vi "View_series_FITS.vi"() -> ()   [LabVIEW 2017] (continued)
, 109.0, 70.0, 62.0, 60.0, 158.0, 79.0, 92.0, 161.0, 66.0, 67.0, 78.0, 96.0, 109.0, 51.0, 173.0, 108.0, 147.0, 183.0, 74.0, 94.0, 120.0, 80.0, 134.0, 89.0, 56.0, -16.0, 94.0, 90.0, 26.0, 124.0, 88.0, 88.0, 82.0, 56.0, 67.0, 93.0, 104.0, 82.0, 121.0, 84.0, 115.0, 46.0, 101.0, 77.0, 20.0, 108.0, 66.0, 88.0, 74.0, 66.0, 126.0, 130.0, 33.0, 104.0, 88.0, 129.0, 93.0, 91.0, 78.0, 31.0, 129.0, 73.0, 40.0, 105.0, 78.0, 80.0, 99.0, 114.0, 52.0, 108.0, 54.0, 63.0, 88.0, 99.0, 96.0, 116.0, 92.0, 84.0, 146.0, 71.0, 65.0, 106.0, 107.0, 133.0, 136.0, 109.0, 113.0, 73.0, 41.0, 90.0, 175.0, 81.0, 107.0, 134.0, 135.0, 104.0, 85.0, 121.0, 80.0, 109.0, 166.0, 147.0, 133.0, 117.0, 132.0, 154.0, 125.0, 124.0, 150.0, 200.0, 161.0, 126.0, 171.0, 266.0, 175.0, 177.0, 301.0, 265.0, 149.0, 143.0, 185.0, 299.0, 158.0, 120.0, 119.0, 255.0, 290.0, 245.0, 254.0, 309.0, 205.0, 224.0, 379.0, 343.0, 303.0, 316.0, 480.0, 435.0, 437.0, 410.0, 625.0, 508.0, 572.0, 872.0, 768.0, 1180.0, 1554.0, 1463.0, 1204.0, 1306.0, 1805.0, 1380.0, 1684.0, 1665.0, 2388.0, 1898.0, 1150.0, 1765.0, 1211.0, 1278.0, 1008.0, 755.0, 628.0, 505.0, 380.0, 509.0, 498.0, 455.0, 590.0, 512.0, 447.0, 285.0, 518.0, 373.0, 347.0, 317.0, 322.0, 335.0, 182.0, 205.0, 264.0, 179.0, 156.0, 290.0, 216.0, 180.0, 107.0, 66.0, 97.0, 100.0, 130.0, 148.0, 131.0, 97.0, 112.0, 125.0, 104.0, 157.0, 124.0, 154.0, 66.0, 113.0, 70.0, 83.0, 127.0, 97.0, 133.0, 80.0, 106.0, 69.0, 123.0, 128.0, 87.0, 116.0, 106.0, 124.0, 96.0, 61.0, 112.0, 69.0, 77.0, 43.0, 88.0, 138.0, 109.0, 102.0, 48.0, 56.0, 88.0, 44.0, 80.0, 106.0, 84.0, 59.0, 88.0, 72.0, 115.0, 82.0, 22.0, 57.0, 78.0, 100.0, 84.0, 79.0, 125.0, 91.0, 85.0, 106.0, -2.0, 0.0, -10.0, 1.0, 2.0, 0.0, 12.0, -14.0, 0.0, 186.0, 188.0, 100.0, 148.0, 52.0, 86.0, 80.0, 90.0, 64.0, 98.0, 80.0, 106.0, 102.0, 100.0, 136.0, 90.0, 40.0, 134.0, 74.0, 64.0, 120.0, 74.0, 134.0, 96.0, 62.0, 80.0, 102.0, 106.0, 58.0, 122.0, 100.0, 70.0, 126.0, 74.0, 80.0, 112.0, 44.0, 94.0, 118.0, 80.0, 114.0, 144.0, 86.0, 72.0, 102.0, 128.0, 88.0, 120.0, 94.0, 136.0, 146.0, 122.0, 134.0, 106.0, 160.0, 174.0, 204.0, 276.0, 280.0, 200.0, 334.0, 240.0, 220.0, 342.0, 302.0, 330.0, 250.0, 354.0, 268.0, 258.0, 236.0, 158.0, 194.0, 144.0, 218.0, 134.0, 130.0, 116.0, 80.0, 110.0, 126.0, 130.0, 120.0, 98.0, 130.0, 100.0, 148.0, 106.0, 98.0, 110.0, 128.0, 98.0, 72.0, 104.0, 108.0, 132.0, 104.0, 108.0, 66.0, 204.0, 104.0, 104.0, 114.0, 86.0, 104.0, 38.0, 128.0, 104.0, 100.0, 122.0, 72.0, 72.0, 122.0, 156.0, 140.0, 132.0, 148.0, 86.0, 72.0, 106.0, 122.0, 140.0, 68.0, 82.0, 110.0, 80.0, 130.0, 88.0, 98.0, 112.0, 136.0, 138.0, 224.0, 86.0, 82.0, 104.0, 36.0, 86.0, 82.0, 100.0, 108.0, 108.0, 140.0, 100.0, 162.0, 118.0, 92.0, 100.0, 134.0, 68.0, 114.0, 102.0, 154.0, 84.0, 96.0, 178.0, 116.0, 224.0, 132.0, 78.0, 166.0, 130.0, 142.0, 114.0, 144.0, 84.0, 76.0, 148.0, 278.0, 122.0, 208.0, 172.0, 174.0, 132.0, 82.0, 94.0, 124.0, 202.0, 134.0, 170.0, 176.0, 156.0, 160.0, 130.0, 260.0, 244.0, 164.0, 208.0, 330.0, 324.0, 286.0, 462.0, 460.0, 358.0, 298.0, 422.0, 496.0, 368.0, 356.0, 492.0, 636.0, 582.0, 912.0, 590.0, 728.0, 960.0, 1122.0, 1322.0, 1146.0, 1358.0, 1412.0, 1668.0, 1750.0, 1348.0, 1494.0, 1784.0, 1630.0, 2430.0, 2424.0, 2260.0, 2330.0, 2126.0, 1934.0, 2190.0, 1808.0, 2816.0, 1314.0, 1562.0, 944.0, 1196.0, 1498.0, 1230.0, 1150.0, 930.0, 856.0, 894.0, 738.0, 720.0, 714.0, 570.0, 602.0, 560.0, 482.0, 432.0, 392.0, 480.0, 290.0, 352.0, 378.0, 292.0, 252.0, 352.0, 286.0, 236.0, 280.0, 258.0, 186.0, 266.0, 310.0, 282.0, 212.0, 342.0, 232.0, 222.0, 208.0, 230.0, 174.0, 280.0, 196.0, 138.0, 232.0, 256.0, 132.0, 154.0, 166.0, 262.0, 220.0, 184.0, 130.0, 204.0, 150.0, 124.0, 158.0, 210.0, 190.0, 94.0, 154.0, 146.0, 126.0, 148.0, 110.0, 152.0, 198.0, 152.0, 168.0, 118.0, 80.0, 76.0, 124.0, 150.0, 130.0, 102.0, 122.0, 128.0, 162.0, 136.0, 96.0, 232.0, 154.0, 102.0, 150.0, 102.0, 96.0, 114.0, 118.0, 106.0, 166.0, 118.0, 144.0, 154.0, 200.0, 140.0, 54.0, 112.0, 106.0, 142.0, 108.0, 170.0, 138.0, 122.0, 120.0, 96.0, 92.0, 156.0, 120.0, 196.0, 130.0, 144.0, 138.0, 164.0, 64.0, 200.0, 166.0, 212.0, 162.0, 206.0, 148.0, 134.0, 128.0, 152.0, 180.0, 164.0, 194.0, 180.0, 168.0, 102.0, 146.0, 180.0, 152.0, 228.0, 132.0, 158.0, 126.0, 130.0, 170.0, 130.0, 128.0, 168.0, 92.0, 164.0, 164.0, 96.0, 130.0, 118.0, 104.0, 112.0, 162.0, 184.0, 140.0, 232.0, 68.0, 72.0, 146.0, 108.0, 96.0, 102.0, 114.0, 108.0, 152.0, 132.0, 124.0, 82.0, 126.0, 116.0, 96.0, 128.0, 48.0, 86.0, 96.0, 62.0, 156.0, 126.0, 118.0, 132.0, 150.0, 128.0, 64.0, 54.0, 44.0, 52.0, 76.0, 112.0, 156.0, 120.0, 138.0, 136.0, 128.0, 114.0, 86.0, 80.0, 94.0, 150.0, 110.0, 164.0, 64.0, 110.0, 74.0, 130.0, 114.0, 96.0, 114.0, 166.0, 144.0, 64.0, 98.0, 70.0, 92.0, 102.0, 130.0, 90.0, 82.0, 80.0, 68.0, 166.0, 84.0, 32.0, 100.0, 82.0, 110.0, 144.0, 72.0, 78.0, 208.0, 102.0, 144.0, 96.0, 106.0, 56.0, 96.0, 110.0, 82.0, 68.0, 112.0, 168.0, 124.0, 124.0, 42.0, 78.0, 114.0, 82.0, 134.0, 142.0, 122.0, 124.0, 84.0, 116.0, 96.0, 86.0, 106.0, 70.0, 92.0, 124.0, 142.0, 144.0, 80.0, 84.0, 70.0, 106.0, 152.0, 92.0, 50.0, 110.0, 90.0, 100.0, 98.0, 110.0, 82.0, 78.0, 94.0, 80.0, 88.0, 90.0, 90.0, 46.0, 86.0, 122.0, 60.0, 65.0, 120.0, 78.0, 80.0, 77.0, 88.0, 124.0, 98.0, 163.0, 94.0, 140.0, 84.0, 86.0, 152.0, 73.0, 111.0, 73.0, 77.0, 103.0, 96.0, 91.0, 163.0, 90.0, 96.0, 172.0, 94.0, 130.0, 88.0, 119.0, 47.0, 82.0, 135.0, 116.0, 84.0, 148.0, 68.0, 121.0, 57.0, 162.0, 95.0, 105.0, 51.0, 67.0, 108.0, 102.0, 210.0, 68.0, 109.0, 136.0, 50.0, 188.0, 188.0, 146.0, 132.0, 106.0, 111.0, 56.0, 113.0, 101.0, 108.0, 79.0, 134.0, 89.0, 102.0, 111.0, 92.0, 140.0, 120.0, 56.0, 112.0, 147.0, -31.0, 104.0, 125.0, 15.0, 104.0, 84.0, 77.0, 104.0, 52.0, 121.0, 145.0, 78.0, 125.0, 158.0, 120.0, 78.0, 129.0, 115.0, 102.0, 104.0, 96.0, 151.0, 107.0, 80.0, 108.0, 114.0, 144.0, 69.0, 100.0, 114.0, 137.0, 76.0, 137.0, 66.0, 148.0, 56.0, 156.0, 142.0, 121.0, 130.0, 135.0, 164.0, 120.0, 93.0, 153.0, 116.0, 121.0, 136.0, 90.0, 93.0, 115.0, 44.0, 141.0, 95.0, 96.0, 132.0, 144.0, 209.0, 99.0, 70.0, 128.0, 143.0, 62.0, 141.0, 140.0, 70.0, 107.0, 50.0, 63.0, 151.0, 118.0, 151.0, 71.0, 101.0, 83.0, 109.0, 111.0, 158.0, 86.0, 133.0, 175.0, 154.0, 129.0, 93.0, 76.0, 142.0, 88.0, 38.0, -30.0, 61.0, 117.0, 125.0, 106.0, 86.0, 140.0, 112.0, 165.0, 131.0, 156.0, 132.0, 115.0, 156.0, 146.0, 169.0, 92.0, 111.0, 115.0, 120.0, 116.0, 94.0, 64.0, 80.0, 118.0, 141.0, 43.0, 83.0, 92.0, 132.0, 127.0, 141.0, 119.0, 101.0, 89.0, 92.0, 141.0, 105.0, 141.0, 93.0, 105.0, 95.0, 155.0, 127.0, 85.0, 221.0, 149.0, 131.0, 140.0, 87.0, 56.0, 98.0, 121.0, 23.0, 102.0, 93.0, 101.0, 57.0, 79.0, 116.0, 29.0, 124.0, 63.0, 116.0, 172.0, 101.0, 108.0, 129.0, 121.0, 126.0, 74.0, 78.0, 162.0, 60.0, 78.0, 96.0, 117.0, 103.0, 146.0, 179.0, 256.0, 172.0, 179.0, 39.0, 59.0, 106.0, 77.0, 112.0, 136.0, 133.0, 105.0, 168.0, 166.0, 133.0, 147.0, 172.0, 135.0, 95.0, 76.0, 148.0, 63.0, 145.0, 182.0, 90.0, 107.0, 118.0, 150.0, 84.0, 78.0, 119.0, 158.0, 85.0, 53.0, 160.0, 134.0, 120.0, 134.0, 126.0, 229.0, 125.0, 128.0, 101.0, 132.0, 175.0, 127.0, 202.0, 151.0, 130.0, 108.0, 189.0, 157.0, 112.0, 231.0, 149.0, 193.0, 107.0, 143.0, 151.0, 138.0, 147.0, 123.0, 118.0, 276.0, 96.0, 127.0, 130.0, 151.0, 125.0, 114.0, 119.0, 106.0, 151.0, 129.0, 184.0, 125.0, 89.0, 166.0, 142.0, 133.0, 113.0, 96.0, 143.0, 167.0, 143.0, 216.0, 158.0, 80.0, 216.0, 44.0, 79.0, 123.0, 96.0, 140.0, 153.0, 118.0, 127.0, 119.0, 76.0, 146.0, 97.0, 115.0, 120.0, 129.0, 144.0, 80.0, 105.0, 98.0, 124.0, 111.0, 97.0, 138.0, 124.0, 128.0, 86.0, 113.0, 127.0, 123.0, 128.0, 108.0, 147.0, 108.0, 93.0, 113.0, 59.0, 134.0, 155.0, 108.0, 164.0, 109.0, 127.0, 182.0, 110.0, 180.0, 118.0, 66.0, 88.0, 161.0, 97.0, 175.0, 197.0, 197.0, 157.0, 133.0, 100.0, 130.0, 112.0, 110.0, 200.0, 185.0, 183.0, 144.0, 164.0, 140.0, 114.0, 147.0, 181.0, 267.0, 197.0, 172.0, 157.0, 236.0, 161.0, 209.0, 220.0, 262.0, 210.0, 318.0, 283.0, 173.0, 312.0, 252.0, 237.0, 112.0, 367.0, 343.0, 226.0, 352.0, 311.0, 292.0, 488.0, 539.0, 467.0, 476.0, 430.0, 523.0, 361.0, 558.0, 542.0, 569.0, 788.0, 668.0, 948.0, 709.0, 1137.0, 906.0, 1089.0, 1344.0, 1373.0, 1444.0, 1630.0, 1584.0, 2442.0, 1776.0, 1876.0, 1835.0, 1217.0, 1901.0, 1929.0, 1557.0, 1665.0, 1196.0, 1374.0, 1362.0, 1216.0, 1006.0, 1012.0, 1299.0, 1141.0, 654.0, 905.0, 969.0, 719.0, 570.0, 635.0, 485.0, 693.0, 490.0, 414.0, 377.0, 321.0, 370.0, 372.0, 263.0, 284.0, 197.0, 143.0, 267.0, 263.0, 247.0, 202.0, 293.0, 241.0, 242.0, 147.0, 142.0, 184.0, 191.0, 164.0, 151.0, 160.0, 115.0, 127.0, 178.0, 180.0, 105.0, 221.0, 139.0, 71.0, 130.0, 146.0, 111.0, 93.0, 148.0, 56.0, 56.0, 104.0, 75.0, 113.0, 65.0, 5.0, -8.0, 9.0, -1.0]
  in  "pattern (all files)":string="*.fits"
  in  "path":path=path "C:/DATA/20110304/series_focus_IN_150um"
  out "Input File:":path=path "C:/DATA/20110304/series_focus_IN_150um/111030412.5622.fits"
  out "Image":dbl[][](graph)
  # "A1"
  # "RIGHT"
  # "TOP"
  # "A2"
  # "A3"
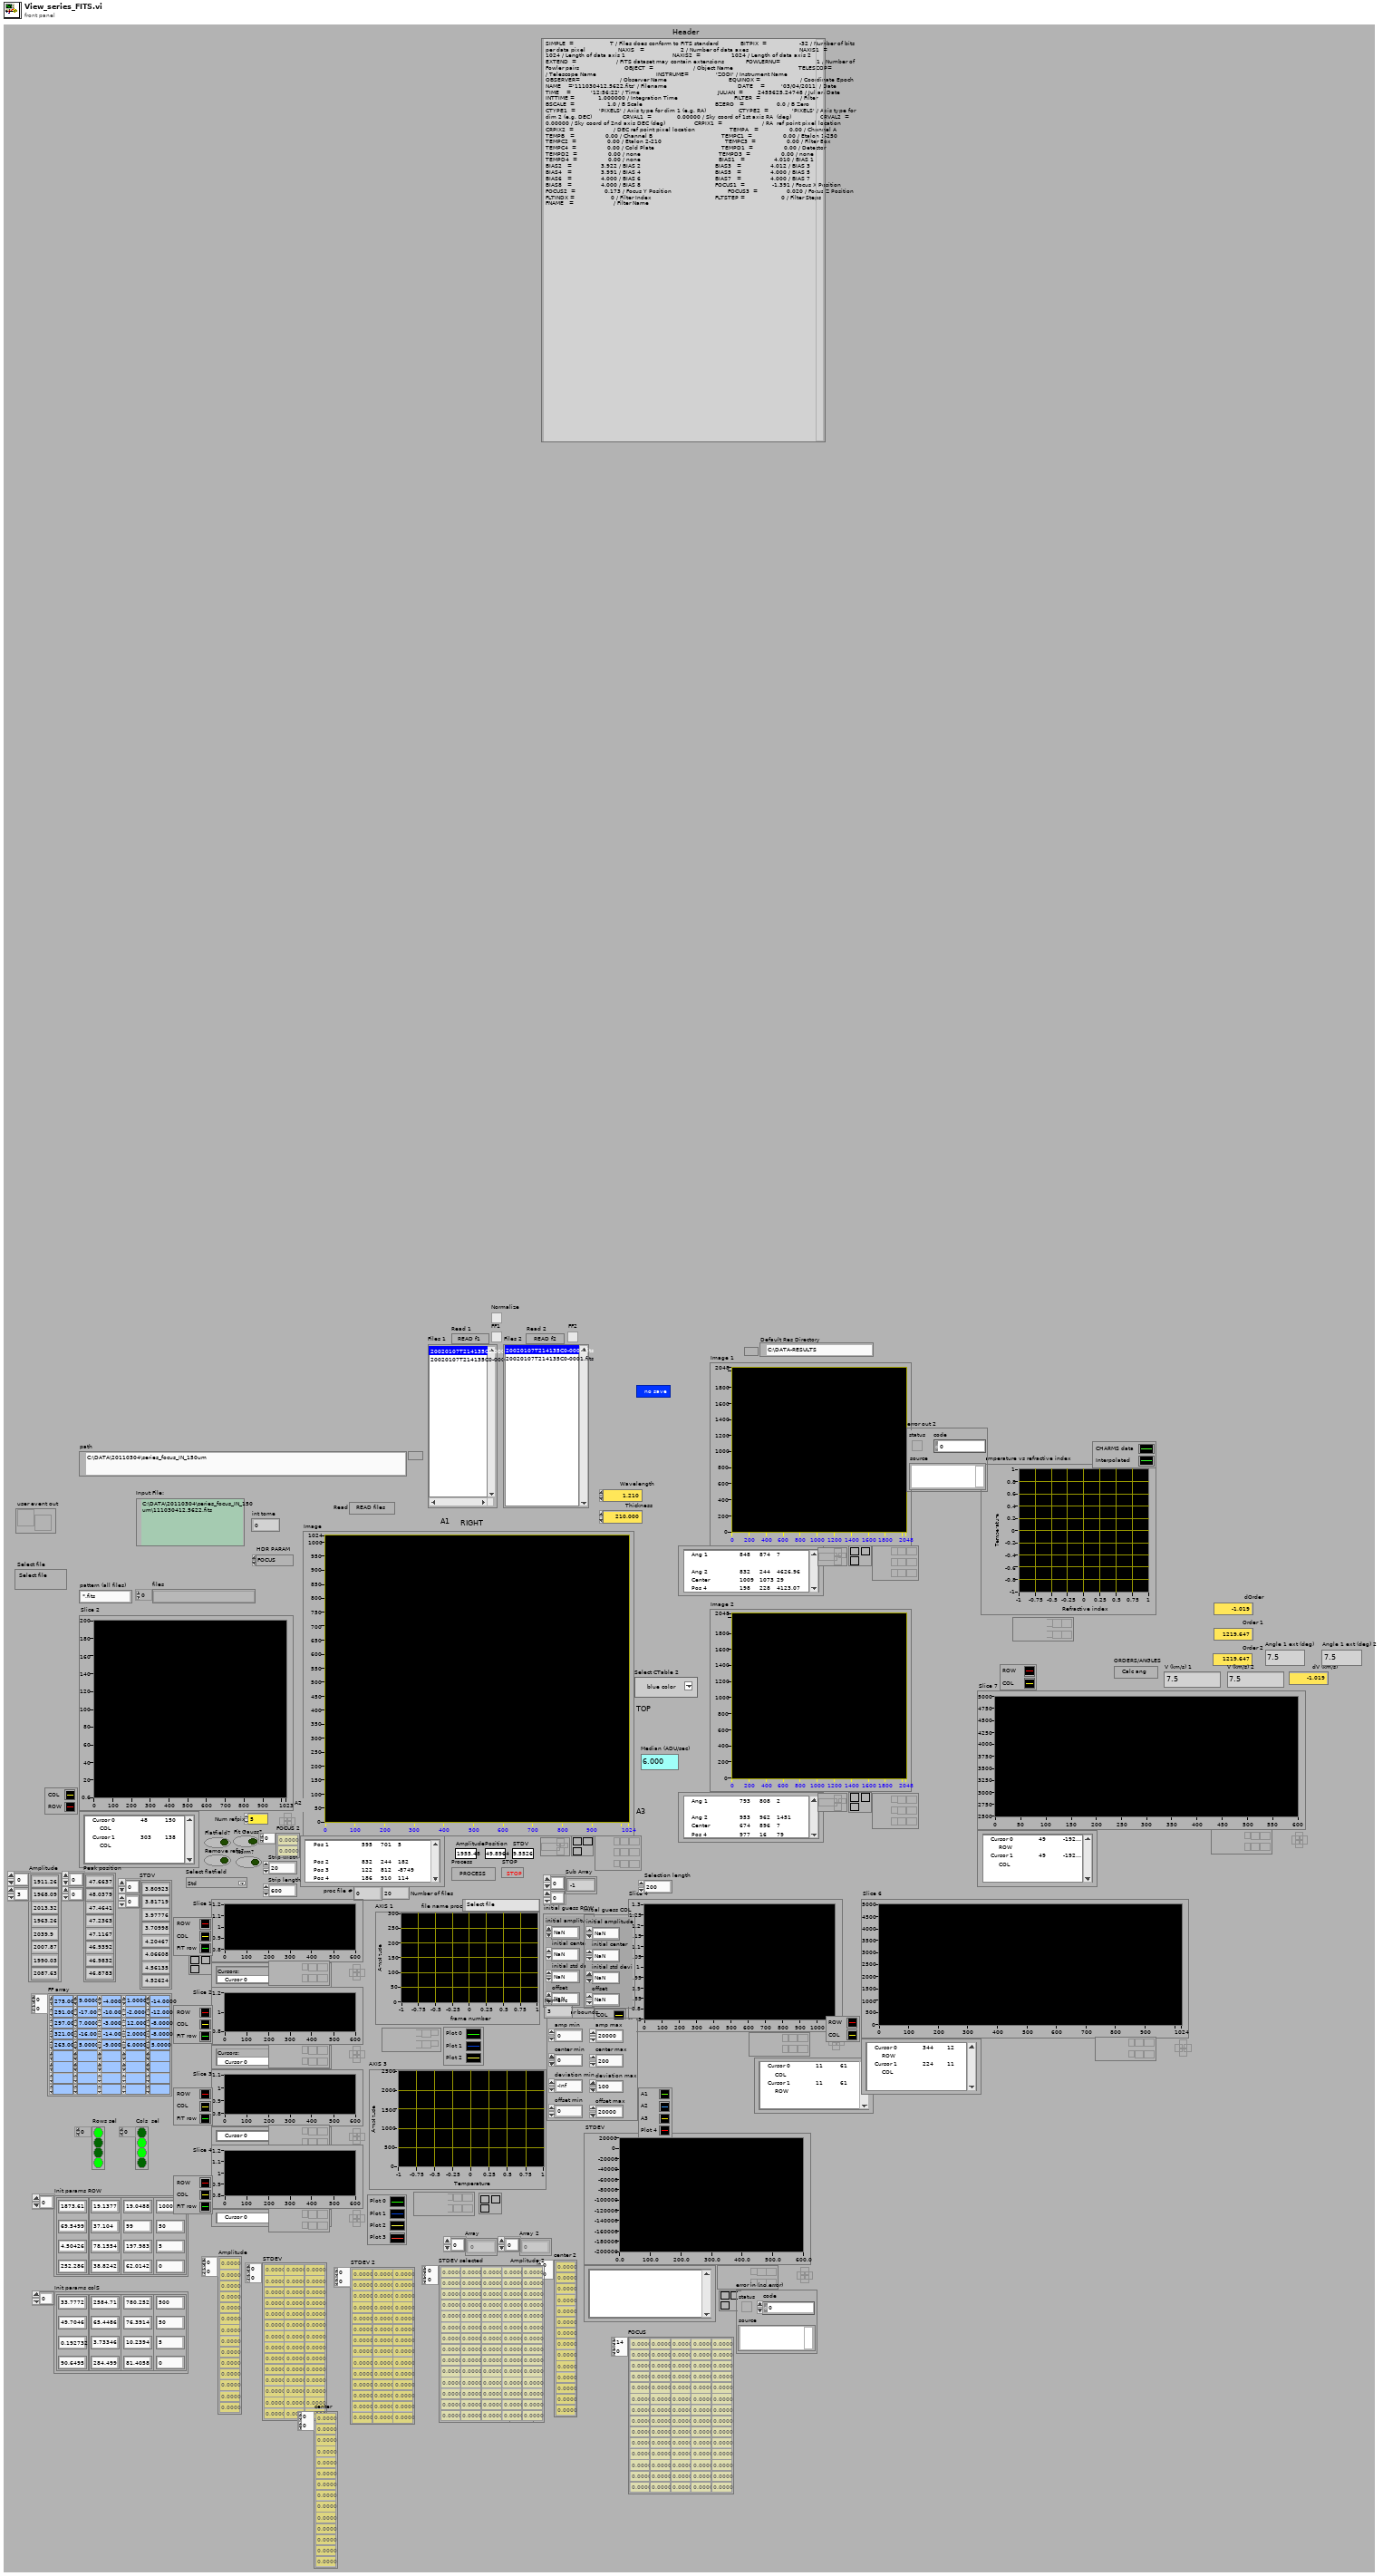
[diagram p1: front panel]
types:
  T1 = typedef "Color Table .ctl" = u16
  T2 = cluster{"initial amplitude":dbl, "initial center":dbl, "initial std devi":dbl, "offset":dbl}[]
  T3 = cluster{"initial amplitude":dbl, "initial center":dbl, "initial std devi":dbl, "offset":dbl}
  T4 = cluster{"amp min":dbl, "amp max":dbl, "center min":dbl, "center max":dbl, "deviation min":dbl, "deviation max":dbl, "offset min":dbl, "offset max":dbl}
  T5 = typedef "RIMAS Control Configuration.ctl" = cluster{"password":string, "Thermal Settings":T6, "Detector Config":T7, "Filter Wheel Config":T10}
  T6 = typedef "Thermal Control Configuration.ctl" = cluster{"Port":refnum<visa-resource-name>, "Recording Interval":dbl}
  T7 = typedef "RIMAS Detector Config.ctl" = cluster{"Detector":u16, "Offsets 0":u16[], "Detector Computer":T8, "FITS hdr template0":path, "FITS hdr template1":path, "FITS Data File Path":path, "FITS Detector Settings":T9, "Offsets 1":u16[]}
  T8 = typedef "RIMAS Detector Server Config.ctl" = cluster{"Machine":string, "Port":u16, "Password":string, "FITS File Path":string, "Header Path":string}
  T9 = typedef "RIMAS Observation Config.ctl" = cluster{"Exp Time Short":dbl, "# of Frames":dbl, "Exp Time Long":dbl, "# of Groups":dbl, "Object Name":string, "Object":string, "Obs Type":string, "Image Type":string, "Observer":string, "Observer Affiliation":string}
  T10 = typedef "RIMAS Filter Wheel Configuration.ctl" = cluster{"Port":refnum<visa-resource-name>, "Filters":T11, "Move parameters":T16, "Steps to move to filters CW":u16[], "delay before \nstop (ms)":u32}
  T11 = typedef "RIMAS Filter Wheel Positions Cluster.ctl" = cluster{"Filter 1":T12, "Filter 2":T13, "FP Filter":T14, "Slit":T15}
  T12 = typedef "RIMAS Filter Wheel enum Filter 1.ctl" = enum16{"H", "K", "Open", "Closed", "Low Res", "Hi Res"}
  T13 = typedef "RIMAS Filter Wheel enum Filter 2.ctl" = enum16{"Y", "J", "Open", "Closed", "Low Res", "Hi Res"}
  T14 = typedef "RIMAS Filter Wheel enum Focal Plane.ctl" = enum16{"H", "K", "Open", "Closed", "Low Res", "Hi Res"}
  T15 = typedef "RIMAS Filter Wheel enum Slit.ctl" = enum16{"0.6 arcSec", "0.8 arcSec", "1.2 arcSec", "3-Open", "4-Open", "5-Open"}
  T16 = typedef "RIMAS Filter Wheel cluster Motor Settings.ctl" = cluster{"MOTOR NUMBER":u8, "Direction":bool, "NUMBER OF  STEPS":u32, "SPEED STEPS/SEC":u16, "ACC/DECEL STEPS/SEC^2":u16, "Move mode":u16}
  T17 = typedef "RIMAS cluster Script Step.ctl" = cluster{"action":T18, "parameter":variant}
  T18 = typedef "RIMAS enum Script Action.ctl" = enum16{"Noop", "Acquire Images", "Move Filter Wheel", "Move Telescope", "Focus", "Wait", "Ask"}
  T19 = cluster{"state":refnum<user-event>, "config":T5, "filter wheel q":refnum<queue>, "vi reference":refnum<vi>, "thermal q":refnum<queue>, "detector q":refnum<queue>, "Det Commands":string[], "Script Notifier":refnum<notifier>, "script":T17[], "script file":path}
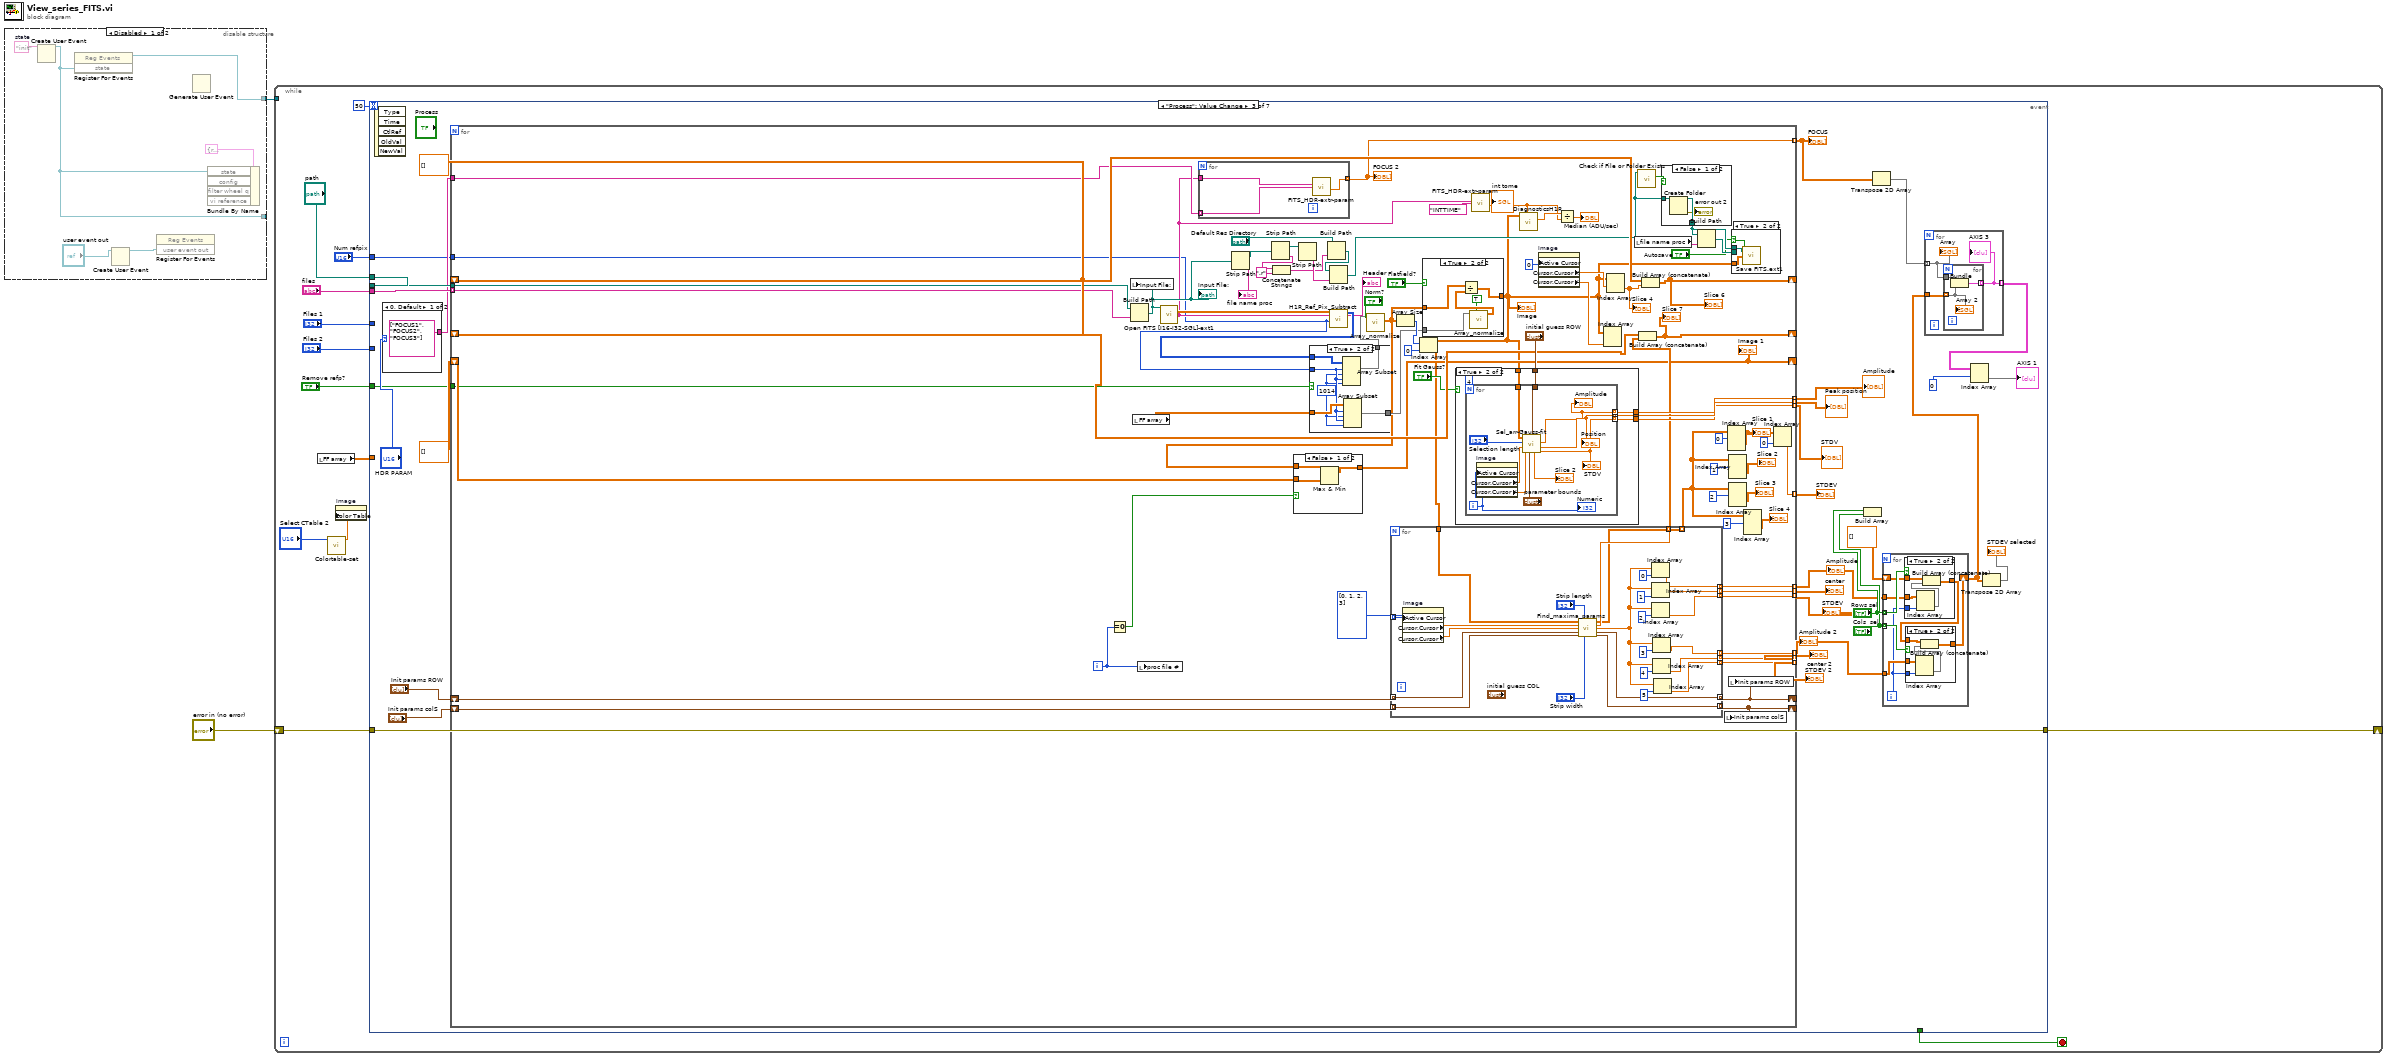
[diagram p0: block diagram]
diagram:
  n1 = disable-structure shown="Disabled" {
    disable-tunnel: [w6 _] -> w1
    disable-tunnel: [w3 _] -> _
    frame Disabled {
      w7 = "init"  # state
      n2 = Create User Event(user event datatype=w7) -> (user event=w3:refnum<user-event>)  [unwired: 1 in, 1 out]
      n3 = register-events(w3) -> (reference out=w6:refnum<event-registration>)  [unwired: 2 in, 1 out]
      n4 = Create User Event(user event datatype="user event out") -> (user event=w8:refnum<user-event>)  [unwired: 1 in, 1 out]
      n5 = register-events(w8) -> ()  [unwired: 2 in, 2 out]
      n6 = Generate User Event() -> ()  [unwired: 4 in, 2 out]
      n7 = Bundle By Name(cluster=T19 {"state"=refnum, "config"={"password"="", "Thermal Settings"={"Port"="", "Recording Interval"=0.0}, "Detector Config"={"Detector"=0, "Offsets 0"=[0, 0, 0, 0, 0, 0, 0, 0, 0, 0, 0, 0, 0, 0, 0, 0, 0, 0, 0, 0, 0, 0, 0, 0, 0, 0, 0, 0, 0, 0, 0, 0], "Detector Computer"={"Machine"="192.168.121.11", "Port"=44444, "Password"="", "FITS File Path"="", "Header Path"=""}, "FITS hdr template0"=path "", "FITS hdr template1"=path "", "FITS Data File Path"=path "", "FITS Detector Settings"={"Exp Time Short"=0.0, "# of Frames"=0.0, "Exp Time Long"=0.0, "# of Groups"=0.0, "Object Name"="", "Object"="", "Obs Type"="", "Image Type"="", "Observer"="", "Observer Affiliation"=""}, "Offsets 1"=[0, 0, 0, 0, 0, 0, 0, 0, 0, 0, 0, 0, 0, 0, 0, 0, 0, 0, 0, 0, 0, 0, 0, 0, 0, 0, 0, 0, 0, 0, 0, 0]}, "Filter Wheel Config"={"Port"="", "Filters"={"Filter 1"=enum."H", "Filter 2"=enum."Y", "FP Filter"=enum."H", "Slit"=enum."0.6 arcSec"}, "Move parameters"={"MOTOR NUMBER"=1, "Direction"=TRUE, "NUMBER OF  STEPS"=7700, "SPEED STEPS/SEC"=2000, "ACC/DECEL STEPS/SEC^2"=1000, "Move mode"=0}, "Steps to move to filters CW"=[10000, 7000, 8000, 8000, 7000, 10000], "delay before \nstop (ms)"=8000}}, "filter wheel q"=refnum, "vi reference"=refnum, "thermal q"=refnum, "detector q"=refnum, "Det Commands"=[], "Script Notifier"=refnum, "script"=[], "script file"=path ""}, "state"=w3) -> ()  [unwired: 3 in, 1 out]
    }
    frame Enabled {
    }
  }
  n8 = while {
    shift-right: [w19] -> _
    shift-left: "error in (no error)" -> [w20]
    tunnel: w1 -> [_]
    stop <- w21 stop-if-true
    n9 = local read "FF array"() -> (w11:dbl[][])
    n10 = call <userlib>:"Colortable-set.vi"("Select CTable 2"="Select CTable 2") -> ("Color table out"=w15:dbl[])  [unwired: 10 in]
    n11 = property on="Image" class="IntGraph (strict)"("Color Table"=w15) -> ()  [unwired: 2 in, 2 out]
    n12 = event shown="[2] \"Process\": Value Change" {
      selector: _ -> [_ _ _ _ _ _ _]
      dyn-events: _ -> [_ _ _ _ _ _ _]
      timeout: 50 -> [_ _ _ _ _ _ _]
      tunnel: "path" -> [_ _ w56 w241 _ _ _]
      tunnel: "files" -> [_ _ w55 w242 _ w323 w353]
      tunnel: ["STOP" _ _ _ _ _ _] -> w21
      tunnel: w20 -> [w22 _ w54 w239 _ _ _]
      tunnel: [w22 _ w54 w239 _ _ _] -> w19
      tunnel: "path" -> [_ w25 _ _ _ w324 w352]
      tunnel: "Files 1" -> [_ _ _ _ _ w322 _]
      tunnel: "Files 2" -> [_ _ _ _ _ _ w351]
      tunnel: "Num refpix" -> [_ _ w31 _ _ w317 w346]
      tunnel: w11 -> [_ _ _ _ _ w318 w347]
      tunnel: "Remove refp?" -> [_ _ w30 _ _ w315 w343]
      event Timeout {
        n13 = event-data() -> ()  [unwired: 1 in, 2 out]
      }
      event "Read": Value Change {
        n14 = event-data() -> ()  [unwired: 1 in, 5 out]
        n15 = call "File Dialog"("start path"=w25, "pattern (all files)"="pattern (all files)") -> ("selected path"=w26:path)  [unwired: 10 in, 3 out]
        n16 = List Folder(path=w26) -> (path out=w28:path, filenames=w24:string[])  [unwired: 3 in, 2 out]
        n17 = local write "path"(w28) -> ()
        n18 = property on="Files 2" class="LstBox (strict)"("Item Names"=w24) -> ()  [unwired: 2 in, 2 out]
        n19 = local write "files"(w24) -> ()
        n20 = Array Size(array=w24) -> (size(s)=→"Number of files":i32)
        n21 = property on="Files 1" class="LstBox (strict)"("Item Names"=w24) -> ()  [unwired: 2 in, 2 out]
      }
      event "Process": Value Change {
        w60 = dbl[][] []
        n22 = event-data() -> ()  [unwired: 1 in, 5 out]
        n23 = case shown="0, Default" "HDR PARAM" {
          tunnel: [string[] ["FOCUS1", "FOCUS2", "FOCUS3"] string[] ["TEMPC1", "TEMPC2"]] -> w34
          frame 0, Default {
          }
          frame 1 {
          }
        }
        n24 = for {
          tunnel: w56 -> [w166]
          tunnel: w55 -> [w165] mode=indexing
          tunnel: [w157] -> w57 mode=indexing
          tunnel: [w159] -> w58 mode=indexing
          tunnel: [w158] -> w59 mode=indexing
          shift-right: [w153] -> _
          shift-left: w60 -> [w154]
          shift-right: [w150] -> _
          shift-left: w60 -> [w151]
          tunnel: [w145] -> w36 mode=indexing
          tunnel: [w144] -> w53 mode=indexing
          tunnel: [w142] -> w49 mode=indexing
          tunnel: [w141] -> w37 mode=indexing
          tunnel: [w140] -> w52 mode=indexing
          tunnel: [w139] -> w48 mode=indexing
          shift-right: [w135] -> _
          shift-left: "Init params ROW" -> [w137]
          shift-right: [w134] -> _
          shift-left: "Init params colS" -> [w136]
          tunnel: [w117] -> w43 mode=indexing
          tunnel: w34 -> [w123]
          shift-right: [w118] -> _
          shift-left: dbl[][] [] -> [w119]
          tunnel: [w113] -> w32 mode=indexing
          tunnel: w31 -> [w105]
          tunnel: w30 -> [w104]
          i -> [w116]
          n25 = Equal To 0?(x=w116) -> (x = 0?=w164:bool)
          n26 = Build Path(base path=w166, name or relative path=w165) -> (appended path=w112:path)
          "Input File:" <- w112
          n27 = local write "Input File:"(w112) -> ()
          n28 = local read "FF array"() -> (w122:dbl[][])
          n29 = local write "proc file #"(w116) -> ()
          n30 = call "Open FITS [I16-I32-SGL]-ext1.vi"("Input File:"=w112) -> ("Image"=w149:sgl[][], "Header"=w110:string)  [unwired: 10 in, 3 out]
          "Header" <- w110
          n31 = for {
            tunnel: w110 -> [w176]
            tunnel: w123 -> [w175] mode=indexing
            tunnel: [w174] -> w117 mode=indexing
            n32 = call <userlib>:"FITS_HDR-extr-param.VI"("Header in"=w176, "Param value to write"=w175) -> ("HDR PARAM Value"=w174:dbl)  [unwired: 6 in, 2 out]
          }
          "FOCUS 2" <- w117
          n33 = Strip Path(path=w112) -> (stripped path=w103:path, name=→"file name proc":string)
          n34 = Strip Path(path=w103) -> (stripped path=w102:path, name=w98:string)
          n35 = Concatenate Strings(w98, ".r" ("string")) -> (w96:string)
          n36 = Strip Path(path=w102) -> (name=w99:string)  [unwired: 1 out]
          n37 = Build Path(base path="Default Res Directory", name or relative path=w96) -> (appended path=w100:path)
          n38 = Build Path(base path=w100, name or relative path=w99) -> (appended path=w94:path)
          n39 = call <userlib>:"H1R_Ref_Pix_Subtract.vi"("Num Ref Pix"=w105, "Orig Array"=w149) -> ("Sub Array"=w128:i32[][])  [unwired: 9 in]
          n40 = case shown="True" w104 {
            tunnel: w128 -> [w178 w184]
            tunnel: w105 -> [_ w181]
            tunnel: [w178 w183] -> w127
            tunnel: w122 -> [w177 w182]
            tunnel: [w177 w179] -> w121
            frame False {
            }
            frame True {
              w180 = 1014 ("index")
              n41 = Array Subset(array=w184, index (row)=w181, length (row)=w180, index (col)=w181, length (col)=w180) -> (w183:i32[][])
              n42 = Array Subset(array=w182, index (row)=w181, length (row)=w180, index (col)=w181, length (col)=w180) -> (w179:dbl[][])
            }
          }
          n43 = call <userlib>:"Array_normalize.vi"("Norm?"="Norm?", "Array"=w127) -> ("Array out"=w120:dbl[][])  [unwired: 9 in]
          n44 = case shown="False" w164 {
            tunnel: w119 -> [w235 _]
            tunnel: [w234 w237] -> w118
            tunnel: w120 -> [w236 w237]
            frame False {
              n45 = Max & Min(x=w236, y=w235) -> (max(x,y)=w234:dbl[][])  [unwired: 1 out]
            }
            frame True {
            }
          }
          "Image 1" <- w118
          n46 = Array Size(array=w120) -> (size(s)=w162:i32[])
          n47 = Index Array(array=w162, index=0) -> ()  [unwired: 1 out]
          n48 = case shown="True" "Flatfield?" {
            tunnel: w120 -> [w228 w233]
            tunnel: [w228 w232] -> w89
            tunnel: w121 -> [_ w229]
            frame False {
            }
            frame True {
              n49 = call <userlib>:"Array_normalize.vi"("Norm?"=TRUE, "Array"=w229) -> ("Array out"=w231:dbl[][])  [unwired: 9 in]
              n50 = Divide(x=w233, y=w231) -> (x/y=w232:dbl[][])
            }
          }
          "Image" <- w89
          n51 = for {
            tunnel: [w195] -> w145 mode=indexing
            tunnel: [w194] -> w144 mode=indexing
            tunnel: [w209] -> w143 mode=indexing
            tunnel: [w193] -> w142 mode=indexing
            tunnel: [w192] -> w141 mode=indexing
            tunnel: [w191] -> w140 mode=indexing
            tunnel: [w190] -> w139 mode=indexing
            tunnel: i32[] [0, 1, 2, 3] -> [w208] mode=indexing
            tunnel: w89 -> [w207]
            tunnel: [w189] -> w135 mode=indexing
            tunnel: [w188] -> w134 mode=indexing
            tunnel: w137 -> [w187] mode=indexing
            tunnel: w136 -> [w186] mode=indexing
            tunnel: [w185] -> _ mode=indexing
            tunnel: [w185] -> w124 mode=indexing
            n52 = property on="Image" class="IntGraph (strict)"("Active Cursor"=w208) -> ("Cursor.Cursor X"=w206:dbl, "Cursor.Cursor Y"=w205:dbl)  [unwired: 2 in, 2 out]
            n53 = call <userlib>:"Find_maxima_params.vi"("Array in"=w207, "Strip length"="Strip length", "Cursor.Cursor X"=w206, "Cursor.Cursor Y"=w205, "initial guess ROW"=w187, "initial guess COL"=w186, "Strip width"="Strip width") -> ("Data and fits"=w185:dbl[][], "Slice"=w209:dbl[], "Params out"=w202:dbl[], "initial guess ROW ADJ 2"=w189:T3, "initial guess col  ADJ"=w188:T3)  [unwired: 4 in]
            n54 = Index Array(array=w202, index=1) -> (element=w194:dbl)
            n55 = Index Array(array=w202, index=0) -> (element=w195:dbl)
            n56 = Index Array(array=w202, index=2) -> (element=w193:dbl)
            n57 = Index Array(array=w202, index=3) -> (element=w192:dbl)
            n58 = Index Array(array=w202, index=4) -> (element=w191:dbl)
            n59 = Index Array(array=w202, index=5) -> (element=w190:dbl)
          }
          n60 = case shown="True" "Fit Gauss?" {
            tunnel: "initial guess ROW" -> [_ w216]
            tunnel: [w210 w215] -> w159
            tunnel: [w210 w214] -> w158
            tunnel: [w210 w213] -> w157
            tunnel: w89 -> [_ w211]
            frame False {